vi "Main.vi"() -> ()   [LabVIEW 2020]
uses:
  System.Windows.Forms
  Global_Variable/Global.vi
  Global_Variable/A180648.vi
  <userlib>/_MGI/Menu Building/MenuTypes/MenuStrip/MGI_MenuStrip.lvclass
  <userlib>/_MGI/Menu Building/MenuItemStatusChange/MGI_MenuItemStatusChange.lvclass
  Libraries/S7/S7.lvlib
panel:
  in  "更换产品":refnum<vi>
  out "传感器码":string
  in  "Result":string[][](table)
  out "状态":string
  out "客户软件版本号":string
  in  "Andon":enum32{"未选择", "缺料报警", "质量报警", "故障报警"}(radio)
  out "PLC":bool
  in  "菜单":refnum<k24>(container)
  out "逆向空载":bool
  out "试验计时":u16
  out "产品编号":string
  out "生产数量":i32
  out "合格数量":i32
  out "userStatus":string caption="用户状态"
  out "userName":string caption="用户名"
  out "connectionMode":string caption="联机类型"
  out "产品型号":string
  out "卡簧检测":bool
  out "拉压力曲线":bool
  out "振动NVH":bool
  out "磨合":bool
  out "备用试验2":bool
  out "传感器特性":bool
  out "电流特性":bool
  out "端铆":bool
  out "提示信息":string
  out "错误":bool
  out "时间字符串":string
  out "日期字符串":string
  out "自动":bool=TRUE
  # "滑移力复测及管柱总成装配台"
  # "试验项目"
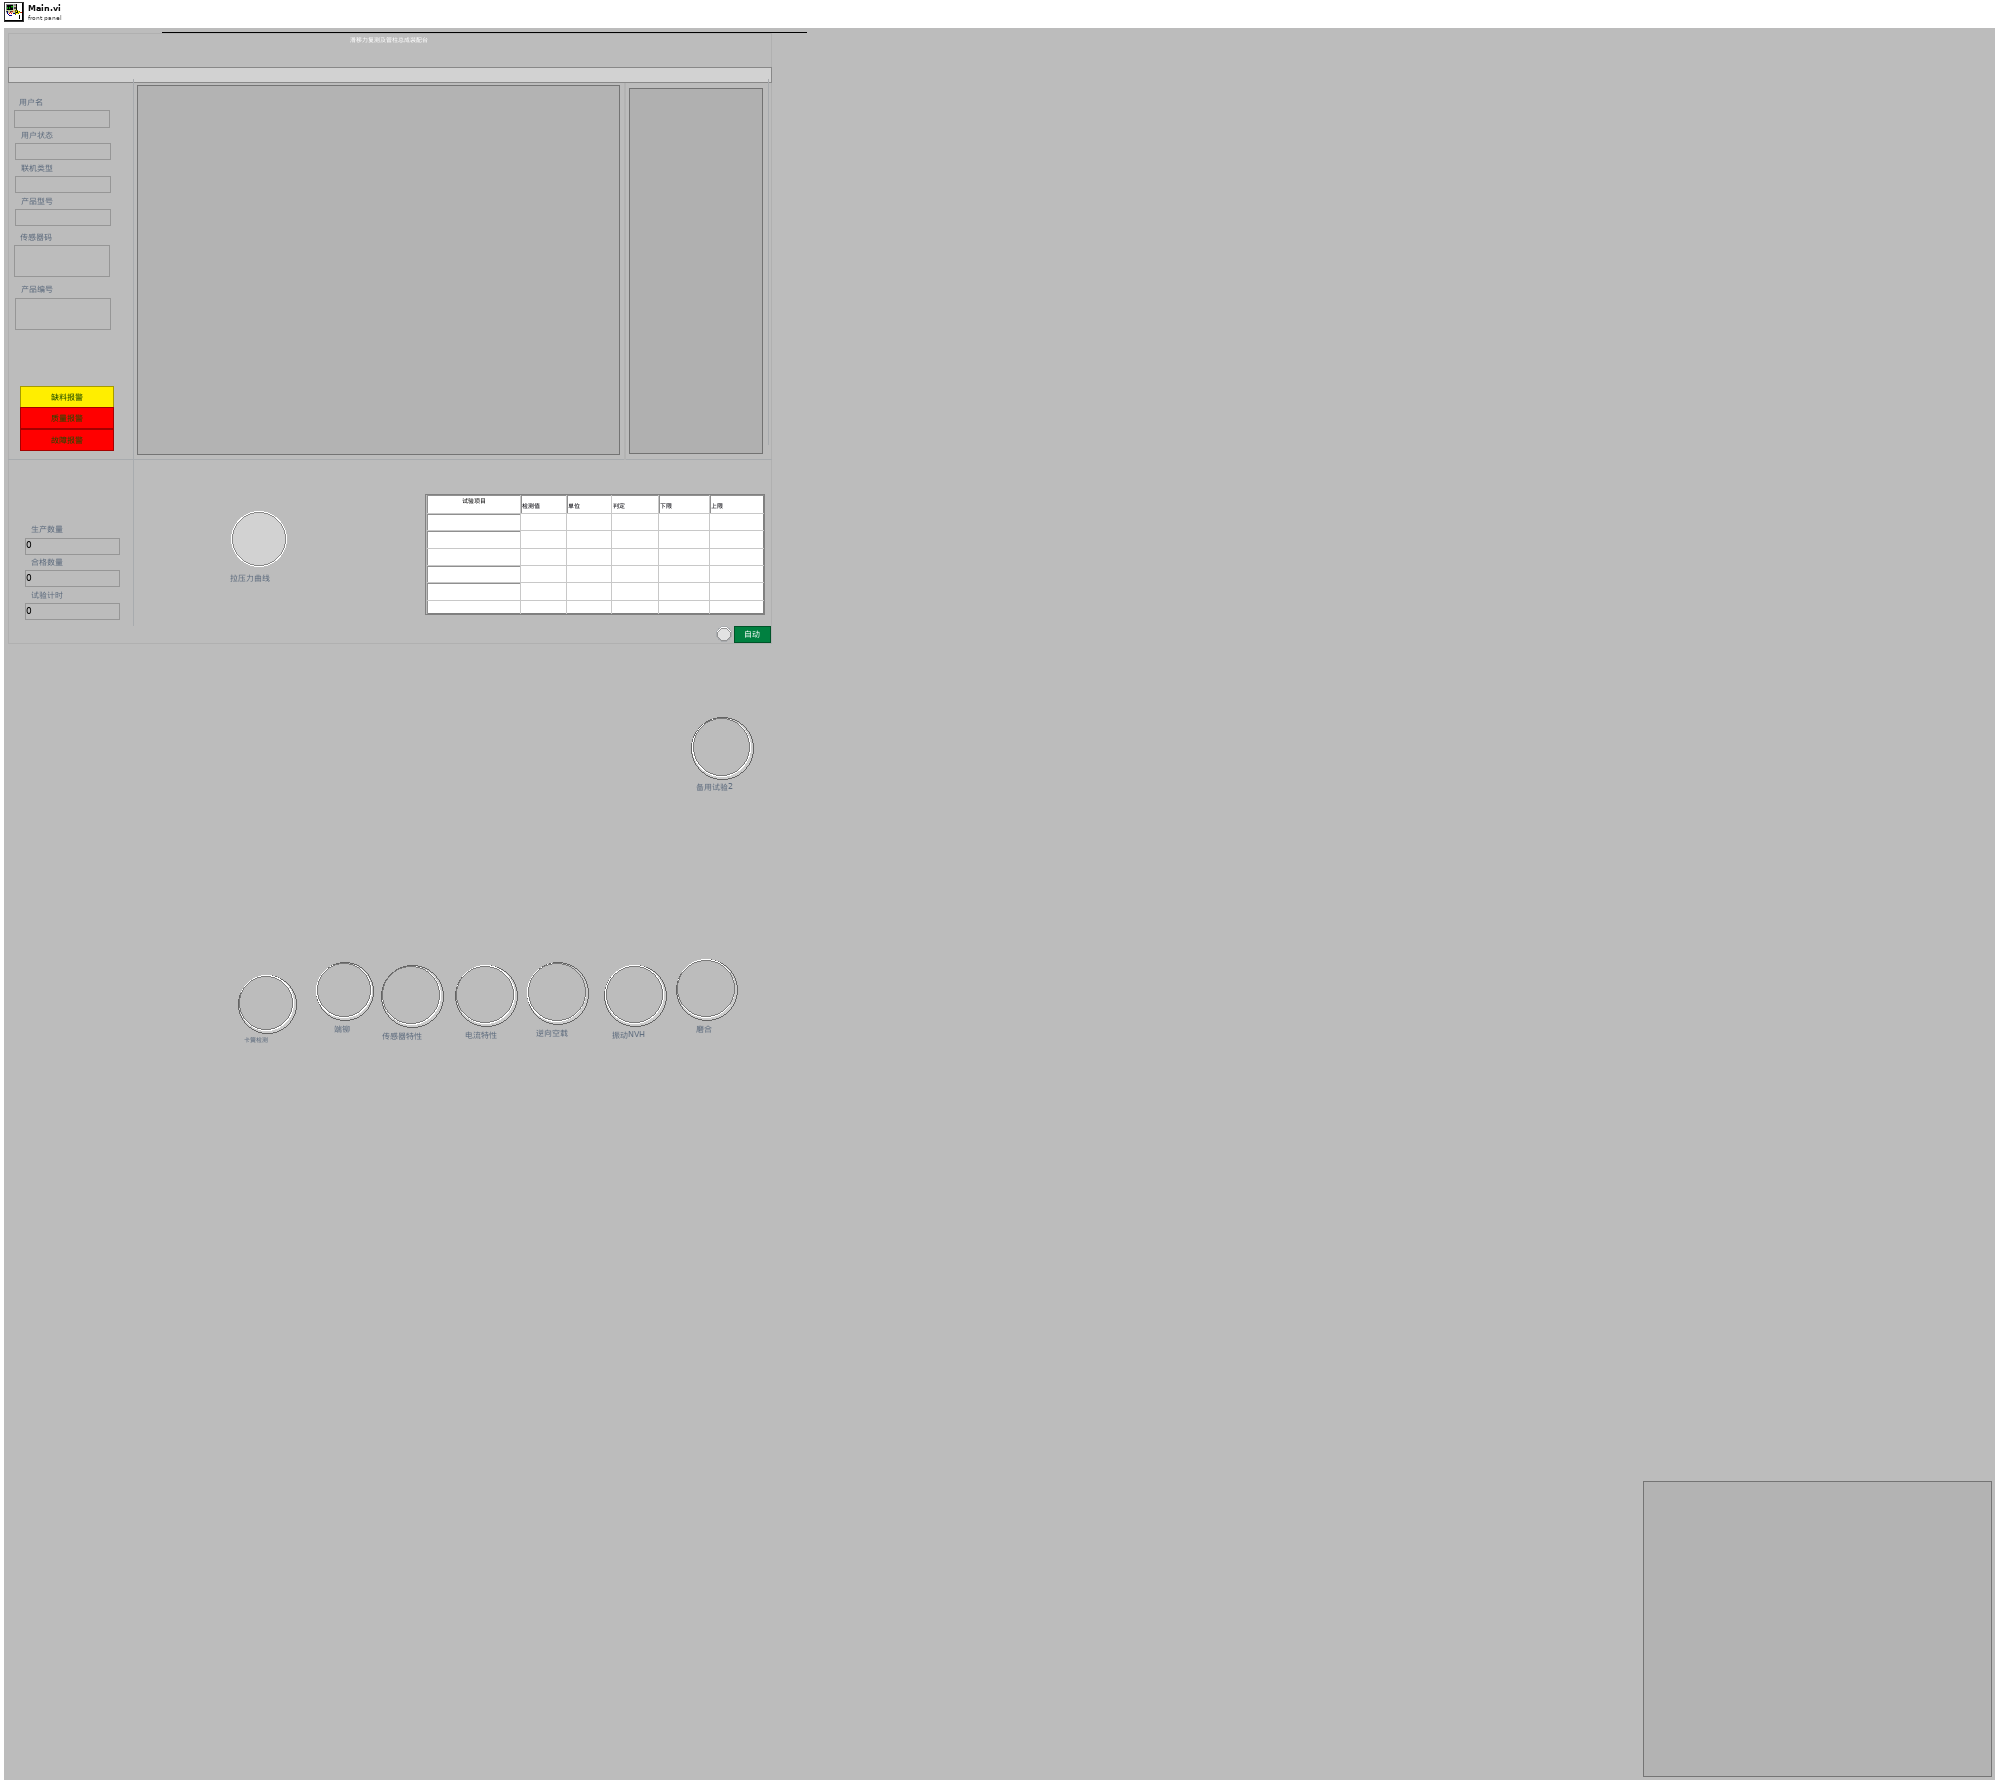
[diagram p1: front panel]
types:
  T1 = typedef "S7.lvlib/Broadcast Events--cluster.ctl" = cluster{"Module Did Init":refnum<user-event>, "Status Updated":refnum<user-event>, "Error Reported":refnum<user-event>, "Module Did Stop":refnum<user-event>, "Update Module Execution Status":refnum<user-event>}
  T2 = enum32{"轴承压装", "侧铆", "端铆", "力特性", "电流特性", "传感器特性", "逆向空载", "磨合"}
  T3 = enum32{"空载", "功能", "力特性", "电流特性", "传感器特性", "逆向空载", "磨合", "振动NVH"}
  T4 = enum32{"Invalid", "Standard", "Closed", "Hidden", "Minimized", "Maximized"}
  T5 = cluster{"设备名称":string, "操作人员":string, "设备状态":enum16{"设备离线", "设备正常", "设备缺料", "设备故障", "质量报警"}, "附加信息":string}
  T6 = enum32{"invalid app kind", "Development System", "Run Time System", "Student Edition", "Embedded LabVIEW", "Evaluation", "Custom"}
  T7 = cluster{"操作员编号":string, "操作员姓名":string, "操作员权限":string, "联机模式":enum16{"单机", "追溯"}}
  T8 = cluster{"Core":cluster{"Current VI Reference":refnum<vi>, "Close Panel on Exit?":bool}, "Your Boolean data":bool, "Your string data":string}
  T9 = cluster{"Current VI Reference":refnum<vi>, "Close Panel on Exit?":bool}
  T10 = cluster{"用户编号":string, "用户名":string, "用户密码(密文)":string, "用户权限":string}
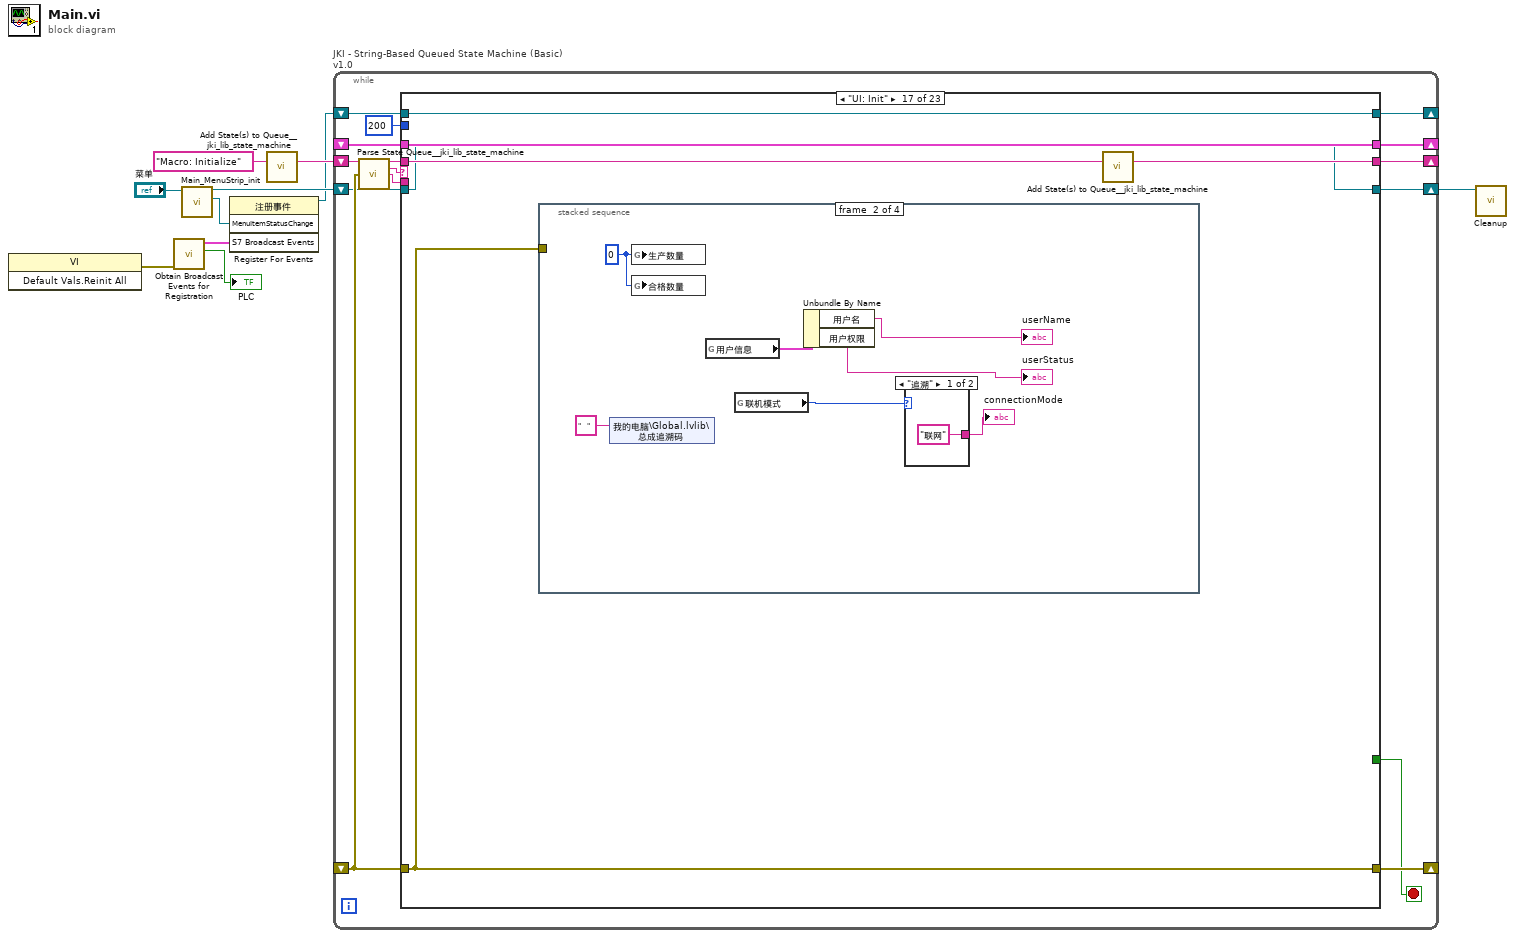
[diagram p0: block diagram]
diagram:
  n1 = invoke class="VI" method="Default Vals.Reinit All"() -> (error out=w3:errorcluster)  [unwired: 3 in, 2 out]
  n2 = call "Obtain Broadcast Events for Registration.vi"("error in (no error)"=w3) -> ("Already running?"=→"PLC":bool, "S7 Broadcast Events"=w5:T1)  [unwired: 8 in, 1 out]
  n3 = call "Main_MenuStrip_init.vi"("MenuStrip"="菜单") -> ("MenuItemStatusChange"=w2:refnum<user-event>, "Menu out"=w7:refnum<class "MGI_MenuStrip.lvclass">)  [unwired: 9 in]
  n4 = register-events(w2, w5) -> (reference out=w1:refnum<event-registration>)  [unwired: 2 in, 1 out]
  n5 = call <vilib>:"Add State(s) to Queue__jki_lib_state_machine.vi"("State(s) in (\"\")"="Macro: Initialize") -> ("States Out"=w10:string)  [unwired: 14 in]
  n6 = while "JKI - String-Based Queued State Machine (Basic) v1.0" {
    shift-right: [w19] -> _
    shift-left: _ -> [w18]
    shift-right: [w21] -> _
    shift-left: _ -> [w16]
    shift-right: [w20] -> _
    shift-left: w10 -> [w22]
    shift-right: [w14] -> w6
    shift-left: w7 -> [w15]
    shift-right: [w12] -> _
    shift-left: w1 -> [w11]
    stop <- w13 stop-if-true
    n7 = call <vilib>:"Parse State Queue__jki_lib_state_machine.vi"("State Queue"=w22, "Error In (no error)"=w16) -> ("Remaining States"=w24:string, "Current State"=w25:string, "Arguments"=w23:string)  [unwired: 11 in]
    n8 = case shown="\"UI: Init\"" w25 {
      selector: w25 -> [_ _ w256 _ _ _ _ _ _ _ _ _ _ _ _ _ _ _ _ _ _ _ _]
      tunnel: w24 -> [w36 w253 w260 w280 w288 w295 w301 w305 w311 w317 w323 w332 w343 w351 w357 w370 w384 w419 w427 w440 w468 w475 w487]
      tunnel: w23 -> [_ _ _ _ _ _ _ _ _ _ _ _ _ _ _ _ _ _ w422 w434 _ _ _]
      tunnel: w18 -> [w34 w250 w258 w271 w285 w293 w298 w306 w314 w320 w326 w329 _ w346 w354 w368 w382 w416 w425 w436 w465 w472 w484]
      tunnel: [w33 w251 w262 w277 errorcluster {"status"=FALSE, "code"=0, "source"=""} ("error out") w292 w299 w303 w309 w316 w322 w330 w340 w347 w355 w361 w380 w417 w423 w437 w466 w473 w485] -> w21
      tunnel: w16 -> [w32 w251 w261 w277 w284 w292 w299 w303 w310 w316 w322 w330 w340 w348 w355 w358 w380 w417 w424 w438 w466 w473 w485]
      tunnel: [w35 w252 w259 w279 w287 w294 w300 w305 w312 w318 w324 w331 w342 w350 w356 w369 w383 w418 w426 w439 w467 w474 w486] -> w20
      tunnel: [w31 w250 w258 w278 w285 w293 w298 w306 w314 w320 w326 w329 w341 w346 w354 w368 w382 w416 w425 w436 w465 w472 w484] -> w19
      tunnel: 200 ("Timeout") -> [w30 _ _ _ _ _ _ _ _ _ _ _ _ _ _ _ _ _ _ _ _ _ _]
      tunnel: w15 -> [w29 w249 w255 w268 w282 w291 w297 w304 w313 w319 w325 w328 w334 w345 w353 w367 w381 w415 w421 w433 w464 w470 w477]
      tunnel: [w28 w249 w255 w268 w282 w291 w297 w304 w313 w319 w325 w328 w334 w345 w353 w367 w381 w415 w421 w433 w464 w470 w477] -> w14
      tunnel: [_ _ _ _ _ TRUE _ _ _ _ _ _ _ _ _ _ _ _ _ _ _ _ _] -> w13
      tunnel: [w26 w248 w254 w267 w281 w289 w296 w307 w308 w315 w321 w327 w335 w344 w352 w366 w379 w412 w420 w432 w463 w469 w476] -> w12
      tunnel: w11 -> [w27 w248 w254 w267 w281 w289 w296 w307 w308 w315 w321 w327 w335 w344 w352 w366 w379 w412 w420 w432 w463 w469 w476]
      frame "", "Event Structure", "Idle" {
        n9 = event shown="[0] 超时" {
          selector: w27 -> [w40 w65 w84 w101 w107 w173 w180 w187 w194 w208 w220 w227 _]
          dyn-events: [w40 w65 w84 w100 w107 w173 w180 w187 w194 w208 w220 w227 _] -> w26
          timeout: w30 -> [_ _ _ _ _ _ _ _ _ _ _ _ _]
          tunnel: w36 -> [w52 w68 w82 w105 w116 w174 w181 w190 w197 w205 w224 w234 w242]
          tunnel: [w51 w67 w81 w105 w114 w175 w182 w191 w198 w206 w225 w233 w242] -> w35
          tunnel: w34 -> [w50 w69 w83 w106 w115 w177 w185 w192 w199 w207 w226 w231 w243]
          tunnel: [w41 w66 w78 w102 w117 w178 w183 w188 w200 w203 w223 w232 w240] -> w33
          tunnel: w32 -> [w41 w66 w79 w103 w117 w178 w183 w188 w201 w203 w223 w232 w240]
          tunnel: [w50 w69 w83 w106 w115 w177 w185 w192 w199 w207 w226 w231 w243] -> w31
          tunnel: w29 -> [w39 _ w80 w104 w110 w176 w184 w189 w196 w204 _ _ w241]
          tunnel: [w39 _ w80 w104 w110 w176 w184 w189 w196 w204 _ _ w241] -> w28
          event Timeout {
            n10 = event-data() -> ()  [unwired: 1 in, 1 out]
            n11 = global read "Global.vi" "计时开始"() -> (w43:bool)
            n12 = global read "Global.vi" "软件版本号"() -> (→"客户软件版本号":string)
            n13 = case shown="真" w43 {
              frame False {
                n14 = global write "Global.vi" "计时复位"(TRUE ("计时复位")) -> ()
              }
              frame True {
                n15 = stacked-sequence {
                  frame #0 {
                    n16 = global read "Global.vi" "计时复位"() -> (w54:bool)
                    n17 = call "已用时间"("Reset"=w54) -> ("Elapsed Time (s)"=→"试验计时":dbl)  [unwired: 11 in, 7 out]
                  }
                  frame #1 {
                    n18 = global write "Global.vi" "计时复位"(FALSE ("计时复位")) -> ()
                  }
                }
              }
            }
            n19 = Format Date/Time String(time format string (%c)="%H:%M ") -> (date/time string=→"时间字符串":string)  [unwired: 2 in]
            n20 = Format Date/Time String(time format string (%c)="%Y年%m月%d日") -> (date/time string=→"日期字符串":string)  [unwired: 2 in]
            n21 = call <vilib>:"Add State(s) to Queue__jki_lib_state_machine.vi"("State(s) in (\"\")"=w52) -> ("States Out"=w51:string)  [unwired: 14 in]
            n22 = global read "Global.vi" "产品编号"() -> (→"产品编号":string)
            n23 = global read "Global.vi" "传感器码"() -> (→"传感器码":string)
            n24 = global read "Global.vi" "合格数量"() -> (→"合格数量":i32)
            n25 = global read "Global.vi" "生产数量"() -> (→"生产数量":i32)
          }
          event "拉压力曲线", "卡簧检测", "端铆", "传感器特性", "电流特性", "振动NVH", "逆向空载", "磨合": Mouse Down {
            w58 = refnum<user-event> refnum items=["轴承压装", "侧铆", "端铆", "力特性", "电流特性", "传感器特性", "逆向空载", "磨合"] ("用户事件输出")
            n26 = event-data() -> ("CtlRef"=w62:refnum<vi>)  [unwired: 1 in]
            n27 = property class="Bool (严格)"(reference=w62) -> ("Label.Text"=w61:string)  [unwired: 1 in, 2 out]
            n28 = vi-ref "Auto.vi"() -> (w64:refnum<vi>)
            n29 = case shown="\"拉力曲线\", 默认" w61 {
              tunnel: [T2."轴承压装" ("试验项目") T2."侧铆" ("试验项目") T2."端铆" ("试验项目") T3."传感器特性" ("事件数据") T3."电流特性" ("事件数据") T3."逆向空载" ("事件数据") T3."振动NVH" ("事件数据") T3."磨合" ("事件数据")] -> w60
              frame "拉力曲线", Default {
              }
              frame "侧铆" {
              }
              frame "端铆" {
              }
              frame "传感器特性" {
              }
              frame "电流特性" {
              }
              frame "逆向空载" {
              }
              frame "振动NVH" {
              }
              frame "磨合" {
              }
            }
            n30 = invoke class="VI" method="Ctrl Val.Get"(reference=w64, "Control Name"="用户事件输出" ("控件名")) -> ("Get Control Value Variant"=w63:variant)  [unwired: 2 in, 3 out]
            n31 = Variant To Data(type=w58, Variant=w63) -> (data=w57:refnum<user-event>)  [unwired: 1 in, 1 out]
            n32 = Generate User Event(user event=w57, event data cluster=w60) -> ()  [unwired: 2 in, 2 out]
            n33 = call <vilib>:"Add State(s) to Queue__jki_lib_state_machine.vi"("State(s) in (\"\")"=w68) -> ("States Out"=w67:string)  [unwired: 14 in]
          }
          event "更换产品": Value Change {
            n34 = event-data() -> ()  [unwired: 1 in, 6 out]
            n35 = vi-ref "Auto.vi"() -> (w91:refnum<vi>)
            n36 = invoke class="VI" method="Ctrl Val.Get"(reference=w91, "Control Name"="产品变更_Event" ("控件名")) -> ("Get Control Value Variant"=w89:variant)  [unwired: 2 in, 3 out]
            n37 = global read "Global.vi" "产品型号"() -> (w85:string)
            n38 = Variant To Data(error in=w79, type=refnum<user-event> refnum ("产品变更_Event"), Variant=w89) -> (data=w87:refnum<user-event>, error out=w86:errorcluster)
            n39 = Generate User Event(user event=w87, event data cluster=w85, error in=w86) -> (error out=w78:errorcluster)  [unwired: 1 in, 1 out]
            n40 = call <vilib>:"Add State(s) to Queue__jki_lib_state_machine.vi"("State(s) in (\"\")"=w82) -> ("States Out"=w81:string)  [unwired: 14 in]
            n41 = local write "产品型号"(w85) -> ()
          }
          event "PLC": Value Change; "PLC": Mouse Down {
            n42 = event-data() -> ()  [unwired: 1 in, 4 out]
            n43 = call "Start Module.vi"("error in (no error)"=w103) -> ("error out"=w94:errorcluster, "Wait for Event Sync?"=w99:bool, "S7 Broadcast Events"=w98:T1, "Module Was Already Running?"=w97:bool)  [unwired: 7 in]
            n44 = local write "PLC"(w97) -> ()
            n45 = register-events(reference=w101, error in=w94, w98) -> (reference out=w100:refnum<event-registration>, error out=w93:errorcluster)  [unwired: 1 in]
            n46 = call "Synchronize Module Events.vi"("error in (no error)"=w93, "Wait for Event Sync?"=w99) -> ("error out"=w92:errorcluster)  [unwired: 9 in]
            n47 = call "Init S7 Link.vi"("error in (no error)"=w92, "超时"=1000, "IP"="192.168.0.71") -> ("error out"=w102:errorcluster)  [unwired: 8 in]
          }
          event User Event {
            n48 = event-data() -> ("StatusChange"=w108:refnum<class "MGI_MenuItemStatusChange.lvclass">)  [unwired: 1 in]
            n49 = call <userlib>:"BasicInfo.vi"("MGI_MenuItemStatusChange in"=w108) -> ("Enabled?"=w111:bool, "Checked?"=w112:bool, "Tag"=w113:string)  [unwired: 7 in, 1 out]
            n50 = case shown="\"退出\"" w113 {
              tunnel: w112 -> [_ _ _ _ _ _ _ _ _ _ _ _ _ _ _]
              tunnel: w111 -> [_ _ _ _ _ _ _ _ _ _ _ _ _ _ _]
              tunnel: [_ _ "S7: Stop\nMacro: Exit" _ _ _ _ _ _ _ _ _ _ _ _] -> w109
              frame "假", Default {
              }
              frame "数据库配置" {
                n51 = global read "用户信息.vi" "用户信息"() -> (w119:T7)
                n52 = Unbundle By Name(w119) -> ("操作员权限"=w118:string)
                n53 = case shown="\"系统管理员\"" w118 {
                  frame Default {
                    n54 = One Button Dialog(message="权限不足！" ("消息")) -> ()  [unwired: 1 in, 1 out]
                  }
                  frame "系统管理员" {
                    n55 = vi-ref "数据库配置.vi"() -> (w122:refnum<vi>)
                    n56 = call "CallVI.vi"("VI引用"=w122, "状态"=T4."Standard") -> ()  [unwired: 12 in, 2 out]
                  }
                }
              }
              frame "退出" {
                n57 = global write "Global.vi" "程序关闭"(TRUE ("程序关闭")) -> ()
                n58 = call "Close_Client.vi"() -> ()  [unwired: 12 in]
              }
              frame "手动控制" {
                n59 = global read "用户信息.vi" "用户信息"() -> (w126:T7)
                n60 = Unbundle By Name(w126) -> ("操作员权限"=w125:string)
                n61 = case shown="\"班组长\", \"系统管理员\"" w125 {
                  frame Default {
                    n62 = One Button Dialog(message="权限不足！" ("消息")) -> ()  [unwired: 1 in, 1 out]
                  }
                  frame "班组长", "系统管理员" {
                    n63 = vi-ref "IO.vi"() -> (w129:refnum<vi>)
                    n64 = call "CallVI.vi"("VI引用"=w129, "状态"=T4."Standard") -> ()  [unwired: 12 in, 2 out]
                  }
                }
              }
              frame "半自动控制" {
                n65 = disable-structure shown="启用" {
                  frame Disabled {
                    n66 = shared-variable "我的电脑\\Global.lvlib\\操作者权限"() -> (w130:string)  [unwired: 1 in, 1 out]
                    n67 = case shown="\"班组长\", \"系统管理员\"" w130 {
                      frame Default {
                        n68 = One Button Dialog(message="权限不足！" ("消息")) -> ()  [unwired: 1 in, 1 out]
                      }
                      frame "班组长", "系统管理员" {
                        n69 = call "CallVI.vi"("VI引用"=refnum<vi> refnum, "状态"=T4."Maximized") -> ()  [unwired: 12 in, 2 out]
                      }
                    }
                  }
                  frame Enabled {
                    n70 = One Button Dialog(message="当前设备不具备半自动功能！" ("消息")) -> ()  [unwired: 1 in, 1 out]
                  }
                }
              }
              frame "产品管理" {
                n71 = vi-ref "Config.vi"() -> (w136:refnum<vi>)
                n72 = call "CallVI.vi"("VI引用"=w136, "状态"=T4."Standard") -> ()  [unwired: 12 in, 2 out]
              }
              frame "系统配置" {
                n73 = global read "用户信息.vi" "用户信息"() -> (w138:T7)
                n74 = Unbundle By Name(w138) -> ("操作员权限"=w137:string)
                n75 = case shown="\"班组长\", \"系统管理员\"" w137 {
                  frame Default {
                    n76 = One Button Dialog(message="权限不足！" ("消息")) -> ()  [unwired: 1 in, 1 out]
                  }
                  frame "班组长", "系统管理员" {
                    n77 = vi-ref "Setting.vi"() -> (w141:refnum<vi>)
                    n78 = call "CallVI.vi"("VI引用"=w141, "状态"=T4."Standard") -> ()  [unwired: 12 in, 2 out]
                  }
                }
              }
              frame "用户管理" {
                n79 = global read "用户信息.vi" "用户信息"() -> (w143:T7)
                n80 = Unbundle By Name(w143) -> ("操作员权限"=w142:string)
                n81 = case shown="\"系统管理员\"" w142 {
                  frame Default {
                    n82 = One Button Dialog(message="权限不足！" ("消息")) -> ()  [unwired: 1 in, 1 out]
                  }
                  frame "系统管理员" {
                    n83 = vi-ref "User_manager.vi"() -> (w146:refnum<vi>)
                    n84 = call "CallVI.vi"("VI引用"=w146, "状态"=T4."Standard") -> ()  [unwired: 12 in, 2 out]
                  }
                }
              }
              frame "编码规则" {
                n85 = global read "用户信息.vi" "用户信息"() -> (w148:T7)
                n86 = Unbundle By Name(w148) -> ("操作员权限"=w147:string)
                n87 = case shown="\"班组长\", \"工艺管理员\", \"系统管理员\"" w147 {
                  frame Default {
                    n88 = One Button Dialog(message="权限不足！" ("消息")) -> ()  [unwired: 1 in, 1 out]
                  }
                  frame "班组长", "工艺管理员", "系统管理员" {
                    n89 = vi-ref "编码规则设置.vi"() -> (w151:refnum<vi>)
                    n90 = call "CallVI.vi"("VI引用"=w151, "状态"=T4."Standard") -> ()  [unwired: 12 in, 2 out]
                  }
                }
              }
              frame "易损件管理" {
                n91 = vi-ref "易损件管理.vi"() -> (w153:refnum<vi>)
                n92 = call "CallVI.vi"("VI引用"=w153, "状态"=T4."Standard") -> ()  [unwired: 12 in, 2 out]
              }
              frame "物料批次管理" {
                n93 = vi-ref "批次管理.vi"() -> (w155:refnum<vi>)
                n94 = call "CallVI.vi"("VI引用"=w155, "状态"=T4."Standard") -> ()  [unwired: 12 in, 2 out]
              }
              frame "报表" {
                n95 = call "文件对话框"("start path"=path "D:/report", "prompt"="打开报表", "pattern (all files)"="*.doc;*.docx", "pattern label"="Word 文档") -> ("selected path"=w156:path, "error out"=w157:errorcluster)  [unwired: 8 in, 2 out]
                n96 = case shown="无错误" w157 {
                  selector: w157 -> [w163 w165]
                  tunnel: w156 -> [w164 _]
                  frame No Error {
                    w162 = 1 items=["Normal", "Maximize", "Minimize"] ("cpubbs_WindowState")
                    n97 = call "Open_Word.vi"("File Path"=w164, "cpubbs_WindowState"=w162, "错误输入（无错误）"=w163) -> ()  [unwired: 12 in, 1 out]
                  }
                  frame Error {
                    n98 = call <vilib>:"Clear Errors.vi"("error in (no error)"=w165) -> ()  [unwired: 5 in, 2 out]
                  }
                }
              }
              frame "报警信息" {
                n99 = vi-ref "报警信息.vi"() -> (w167:refnum<vi>)
                n100 = call "CallVI.vi"("VI引用"=w167, "状态"=T4."Standard") -> ()  [unwired: 12 in, 2 out]
              }
              frame "关于" {
                n101 = vi-ref "About.vi"() -> (w169:refnum<vi>)
                n102 = call "CallVI.vi"("VI引用"=w169, "状态"=T4."Standard") -> ()  [unwired: 12 in, 2 out]
              }
              frame "操作演示" {
                n103 = call <vilib>:"Application Directory.vi"() -> ("Application Directory"=w172:path)
                n104 = Build Path(base path=w172, name or relative path="操作演示" ("名称或相对路径")) -> (appended path=w171:path)
                n105 = call "自动播放ppt.vi"("路径"=w171) -> ()  [unwired: 10 in, 1 out]
              }
            }
            n106 = call <vilib>:"Add State(s) to Queue__jki_lib_state_machine.vi"("State(s) in (\"\")"=w116, "State(s) at Back (\"\")"=w109) -> ("States Out"=w114:string)  [unwired: 13 in]
          }
          event User Event {
            n107 = event-data() -> ("Init?"=w179:bool)  [unwired: 1 in, 1 out]
            n108 = local write "PLC"(w179) -> ()
            n109 = call <vilib>:"Add State(s) to Queue__jki_lib_state_machine.vi"("State(s) in (\"\")"=w174) -> ("States Out"=w175:string)  [unwired: 14 in]
          }
          event User Event {
            n110 = event-data() -> ("Running?"=w186:bool)  [unwired: 1 in]
            n111 = local write "PLC"(w186) -> ()
            n112 = call <vilib>:"Add State(s) to Queue__jki_lib_state_machine.vi"("State(s) in (\"\")"=w181) -> ("States Out"=w182:string)  [unwired: 14 in]
          }
          event User Event {
            n113 = event-data() -> ()  [unwired: 1 in, 7 out]
            n114 = local write "PLC"(FALSE ("PLC")) -> ()
            n115 = call <vilib>:"Add State(s) to Queue__jki_lib_state_machine.vi"("State(s) in (\"\")"=w190) -> ("States Out"=w191:string)  [unwired: 14 in]
          }
          event User Event {
            n116 = event-data() -> ("Error"=w202:errorcluster)  [unwired: 1 in]
            n117 = Merge Errors(w202, w201) -> (w200:errorcluster)
            n118 = call <vilib>:"Add State(s) to Queue__jki_lib_state_machine.vi"("State(s) in Front (\"\")"="S7: Initialize\nIdle", "State(s) in (\"\")"=w197) -> ("States Out"=w198:string)  [unwired: 13 in]